vi "SMain.vi"() -> ()   [LabVIEW 2011] (continued)
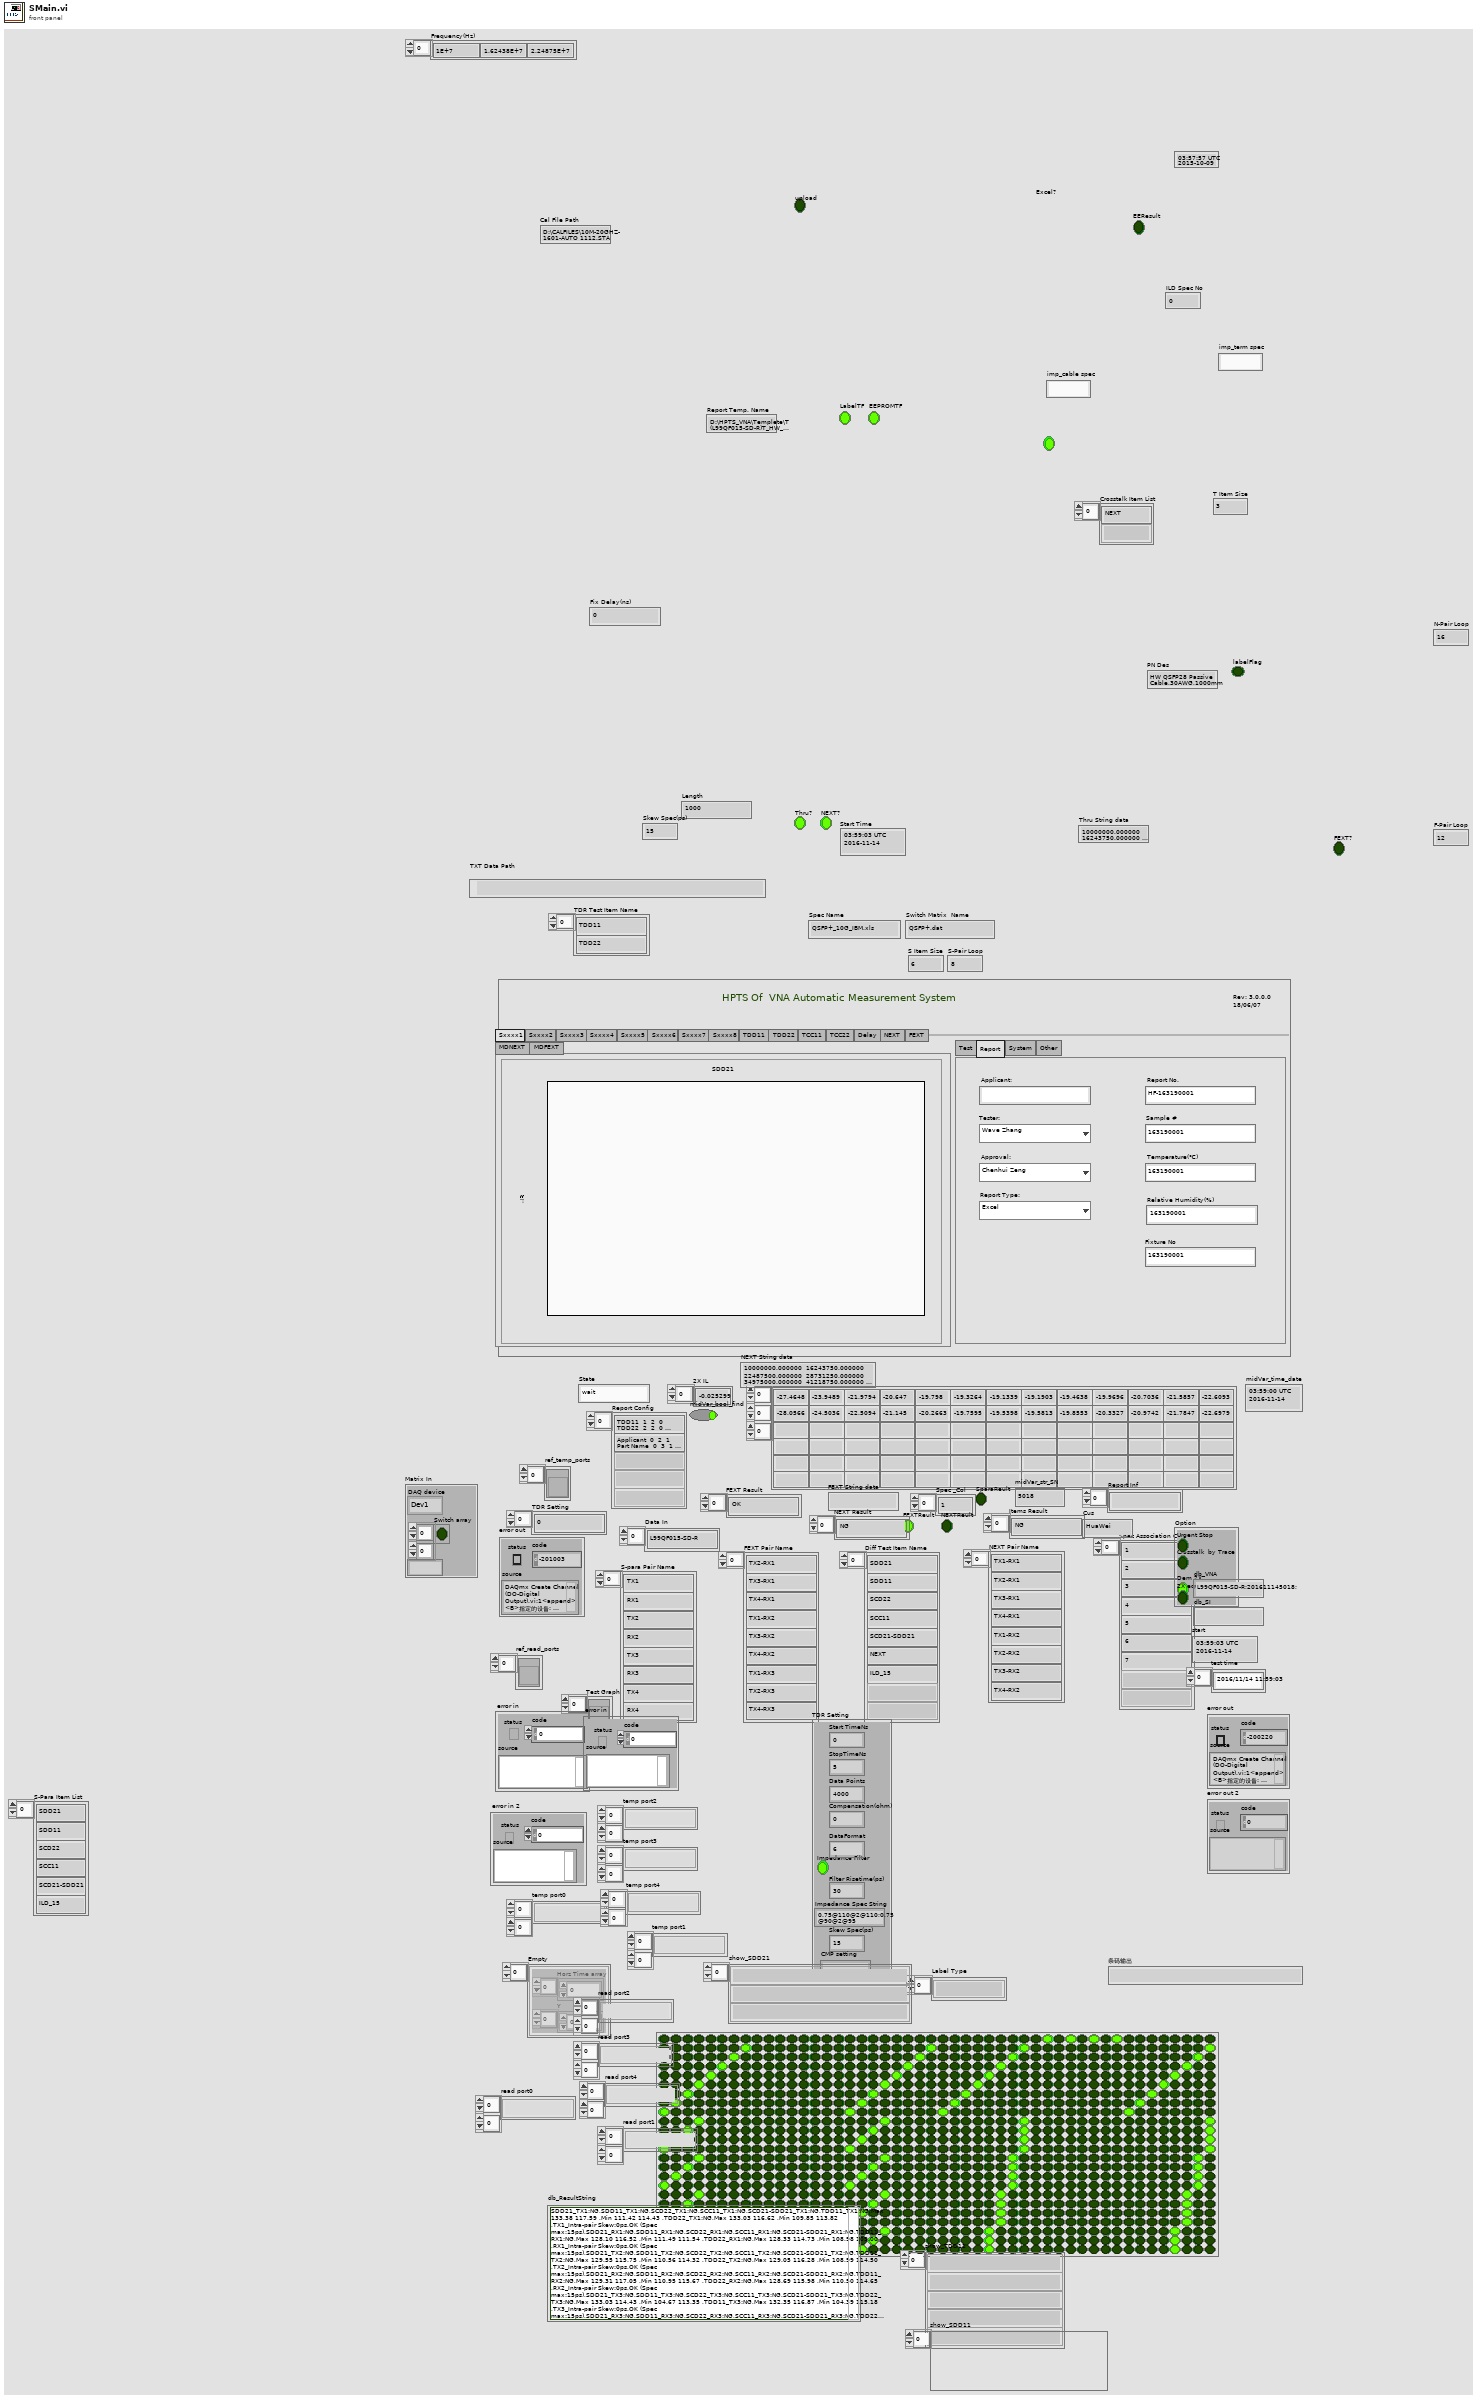
[diagram p1: front panel]
types:
  T1 = typedef "UploadPara.ctl" = cluster{"NetCmdHW":string, "NetPathHW":string, "NetCmdCompress":string, "NetPathCompress1":string, "NetPathCompress2":string, "AlarmDisplay":string, "Synchronous":string, "NetTemppath":string, "NetLocalpath":string}
  T2 = typedef "cluResult.ctl" = cluster{"itemResult":string[], "itemName":string[]}
  T3 = typedef "singleTestParameter.ctl" = cluster{"itemName":string, "testPair":dbl, "chartDisplay?":bool, "spec":cluster{"upper limit":cluster{"dx":dbl[], "dy":dbl[]}, "lowwer limit":cluster{"dx":dbl[], "dy":dbl[]}}, "smooth":cluster{"smooth?":bool, "smoothPoints":dbl}, "Compensation(ohm)":dbl, "Filter Risetime(ps)":dbl, "singlePoint":string[], "offset":dbl[]}
  T4 = typedef "informationIn.ctl" = cluster{"Sample PN: ":string, "SampleSN:":string, "Sparam Test Item":string[], "S-para Pair Name":string[], "Length":string, "Diff Test Item Name":string[], "Diff Test Item Name smooth":string[], "smooth point":dbl, "limitSpec":string[][], "switchIndexOffset":dbl, "testType":enum16{"Loss", "Next", "Fext"}}
  T5 = cluster{"Tab_Graph":refnum<vi>, "Test Graph":refnum<vi>[], "Test Status:":refnum<vi>, "db_ResultString":refnum<vi>}
  T6 = cluster{"Start TimeNs":dbl, "StopTimeNs":dbl, "Data Points":i32, "Compensation(ohm)":dbl, "DataFormat":i16, "Impedance Filter":bool, "Filter Risetime(ps)":dbl, "Impedance Spec String":string, "Skew Spec(ps)":i32, "CMP Setting":string}[]
  T7 = cluster{"start":i32, "length":i32, "p":i32, "H/L":bool}[]
  T8 = cluster{"Server":string, "DB":string, "PSW":string, "User":string}
  T9 = cluster{"auto get refer point":bool, "width1":i32, "width2":i32, "show_TDD11":string[], "show_TDD22":string[], "test time":string[], "show_impspec":string[], "TestResult":bool[], "FileName":string, "FileVersion":string}
  T10 = cluster{"Start TimeNs":dbl, "StopTimeNs":dbl, "Data Points":i32, "Compensation(ohm)":dbl, "DataFormat":i16, "Impedance Filter":bool, "Filter Risetime(ps)":dbl, "Impedance Spec String":string, "Skew Spec(ps)":i32, "CMP Setting":string}
  T11 = cluster{"Urgent Stop":bool, "Crosstalk  by Trace":bool, "Dem 2X":bool, "2X equalize ":bool}
  T12 = cluster{"Start TimeNs":dbl, "StopTimeNs":dbl, "Data Points":i32, "Compensation(ohm)":dbl, "DataFormat":i16, "Impedance Filter":bool, "Filter Risetime(ps)":dbl, "Impedance Spec String":string, "Skew Spec(ps)":i32, "CMP setting":string}
  T13 = cluster{"DAQ device":enum16{"Dev1", "Dev2", "Dev3"}, "Switch array ":bool[][], i32}
  T14 = enum16{"NI PCI-6509", "LX MCU", "LX MCU_40G", "LX MCU_40G_HuaWei"}
  T15 = enum32{"Sxxxx1", "Sxxxx2", "Sxxxx3", "Sxxxx4", "Sxxxx5", "Sxxxx6", "Sxxxx7", "Sxxxx8", "TDD11", "TDD22", "TCC11", "TCC22", "Delay", "NEXT", "FEXT", "MDNEXT", "MDFEXT"}
  T16 = enum16{"Standard Report", "HTML", "Word", "Excel"}
  T17 = enum8{"Enabled", "Disabled", "Disabled and Grayed Out"}
  T18 = typedef "HW_xml.ctl" = cluster{"FileVersion":string, "FileName":string, "test time":string[], "original Path":path, "show_impspec":string[], "usedSN":string, "show_Terminal Point":dbl[], "show_Cable Point":dbl[], "sSpec":T3[], "resultCluster":T2, "customerPN":string}
  T19 = enum32{"invalid app kind", "Development System", "Run Time System", "Student Edition", "Embedded LabVIEW", "Evaluation", "Custom"}
  T20 = cluster{"Urgent Stop":bool, "Crosstalk  by Trace":bool, "Dem 2X":bool, "2x equalize ":bool}
  T21 = cluster{"Demo":bool, "Manual":bool, "Urgent Stop":bool}
  T22 = cluster{"DAQ Device":u16, "Switch array ":bool[][], i32}
  T23 = cluster{"Start TimeNs 2":dbl, "StopTimeNs 2":dbl, "Data Points 2":i32, "Compensation(ohm) 2":dbl, "DataFormat":i16, bool, "Filter Risetime(ps) 2":dbl, "Impedance Spec String 2":string, "Skew Spec(ps) 2":i32, string}
  T24 = cluster{"DAQ Device":u16, "Switch array ":bool[][], "S-Pair Loop":i32}
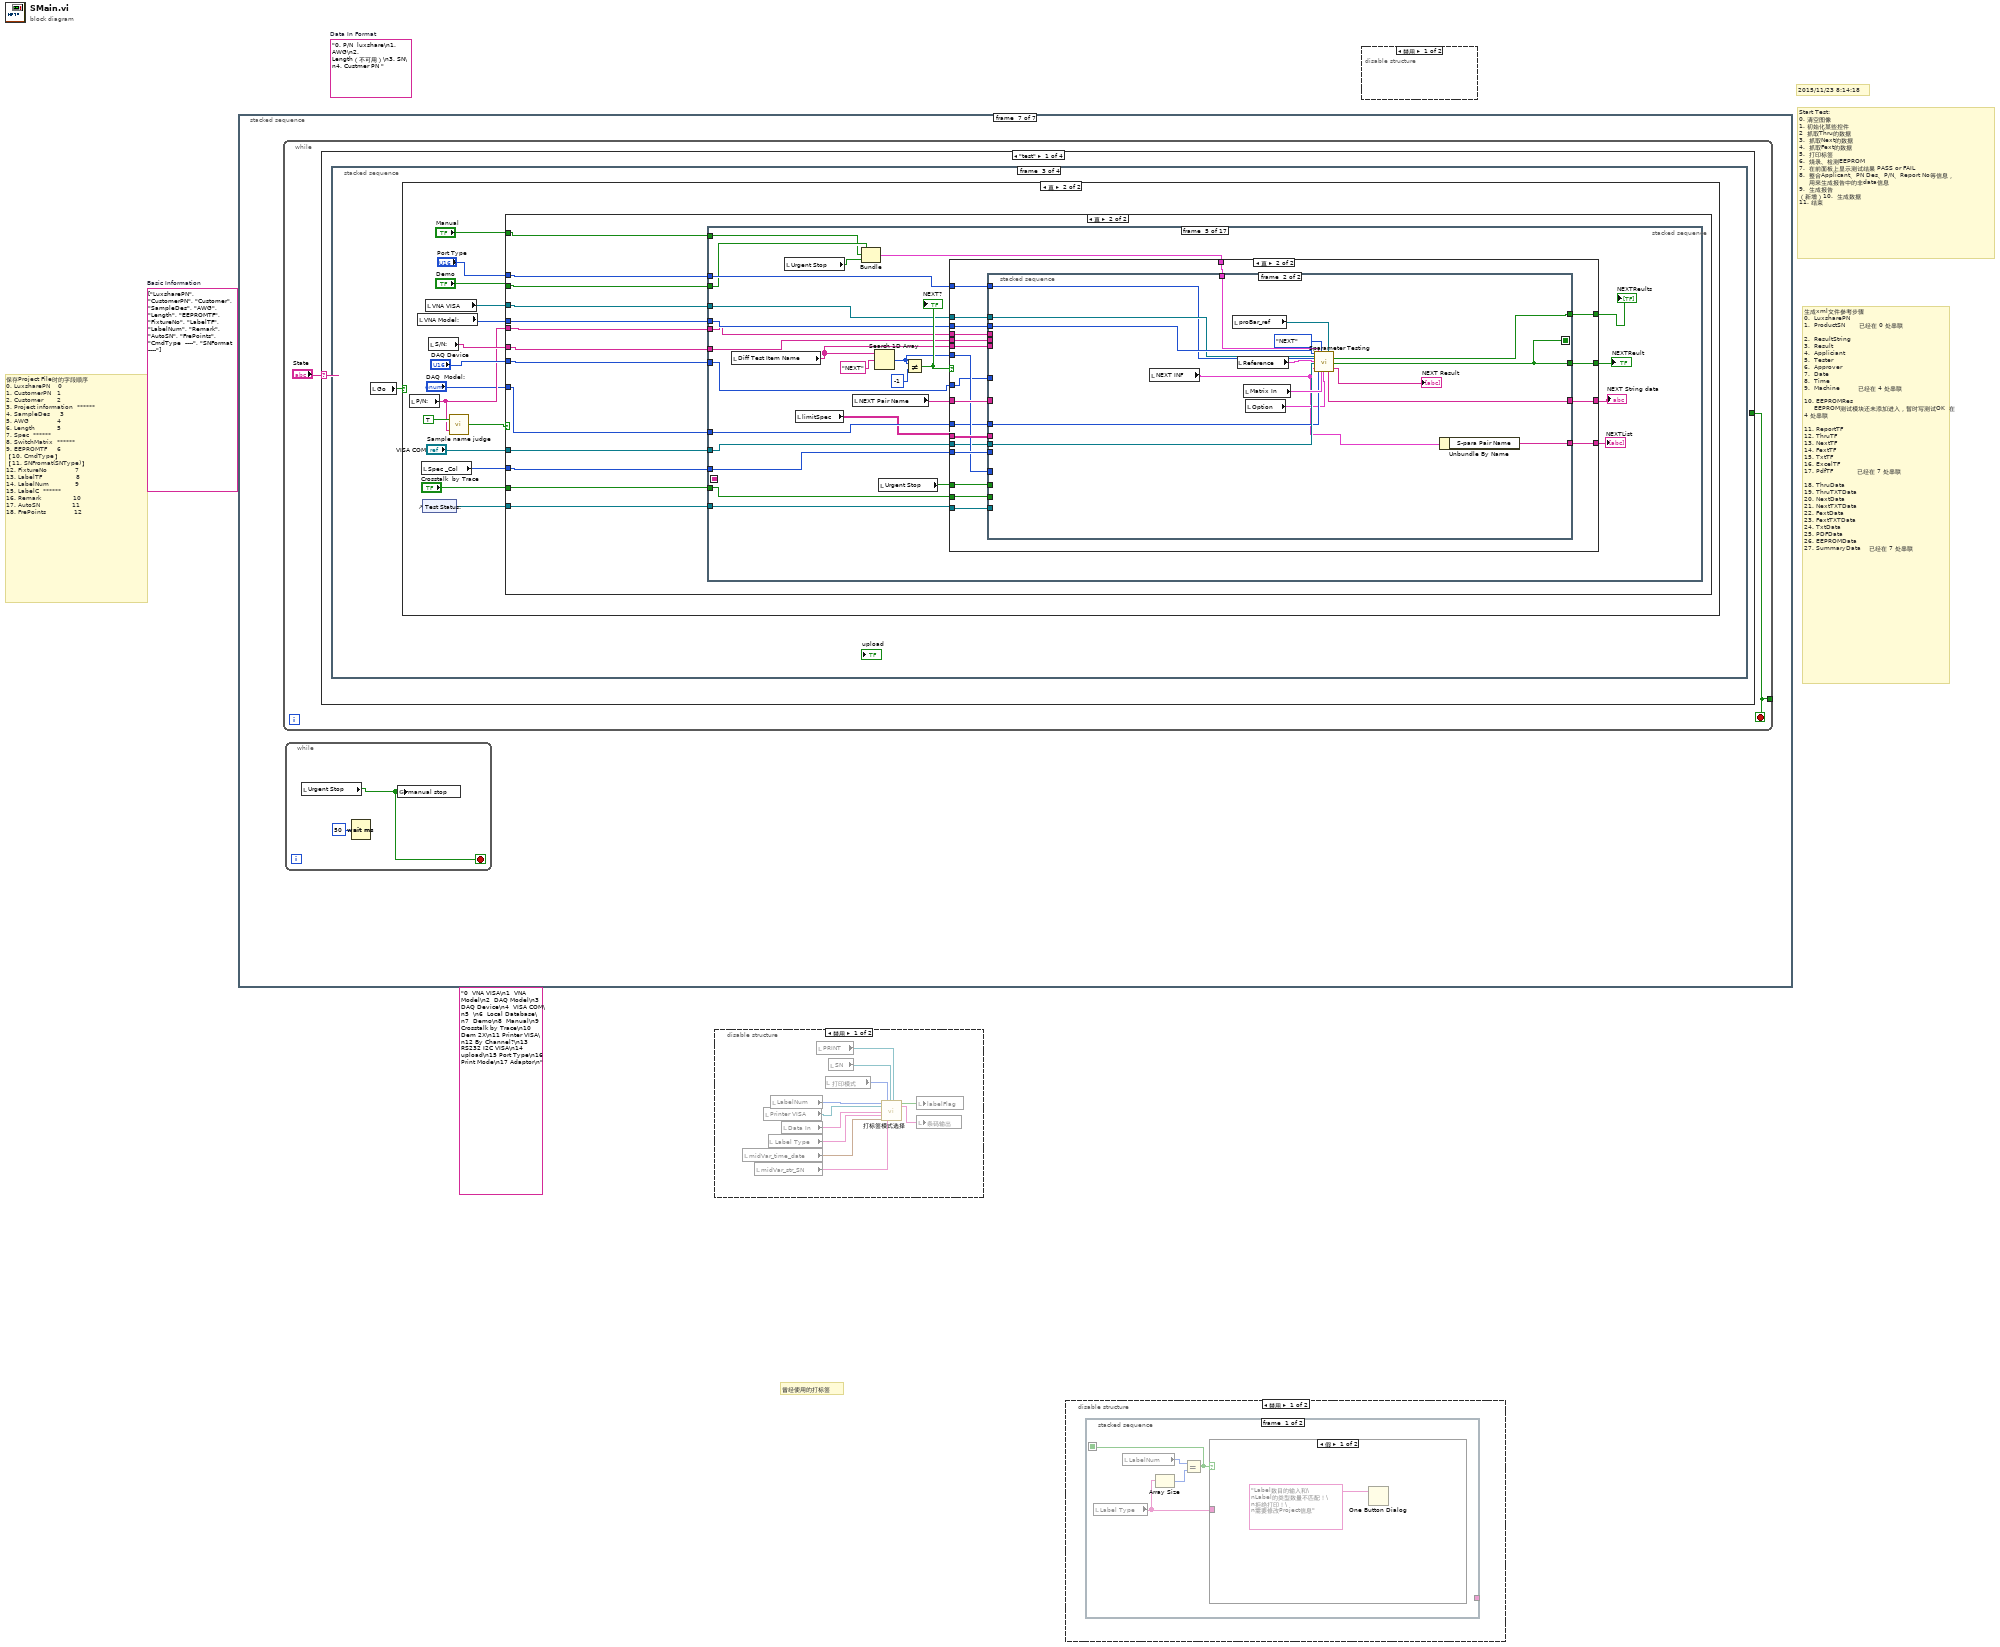
[diagram p0: block diagram]
diagram:
  (unwired) "0  VNA VISA\n1  VNA Model\n2  DAQ Model\n3  DAQ Device\n4  VISA COM\n5  \n6  Local Database\n7  Demo\n8  Manual\n9  Crosstalk by Trace\n10 Dem 2X\n11 Printer VISA\n12 By Channel?\n13 RS232 I2C VISA\n14 upload\n15 Port Type\n16 Print Mode\n17 Adaptor\n"
  (unwired) string[] ["LuxsharePN", "CustomerPN", "Customer", "SampleDes", "AWG", "Length", "EEPROMTF", "FixtureNo", "LabelTF", "LabelNum", "Remark", "AutoSN", "FrePoints", "CmdType  ----", "SNFormat ----"]  # Basic Information
  (unwired) "0. P/N  luxshare\n1. AWG\n2. Length（不可用）\n3. SN\n4. Custmer PN "  # Data In Format
  # "曾经使用的打标签"
  # "保存Project File时的字段顺序\n0. LuxsharePN    0 \n1. CustomerPN   1\n2. Customer       2\n3. Project information  ****** \n4. SampleDes     3\n5. AWG              4\n6. Length           5\n7. Spec  ******\n8. SwitchMatrix  ******  \n9. EEPROMTF     6\n【10. CmdType】           \n【11. SNFromat(SNType)】   \n12. FixtureNo              7\n13. LabelTF                 8\n14. LabelNum             9\n15. LabelC  ******\n16. Remark                10\n17. AutoSN                11\n18. FrePoints              12"
  # "2015/11/23 8:14:18"
  # "生成xml文件参考步骤\n0.  LuxsharePN\n1.  ProductSN       已经在 0 处串联\n\n2.  ResultString     \n3.  Result             \n4.  Appliciant\n5.  Tester\n6.  Approver\n7.  Date \n8.  Time\n9.  Machine         已经在 4 处串联\n\n10. EEPROMRes   \n     EEPROM测试模块还未添加进入，暂时写测试OK  在 4 处串联\n\n11. ReportTF\n12. ThruTF\n13. NextTF\n14. FextTF\n15. TxtTF\n16. ExcelTF\n17. PdfTF            已经在 7 处串联\n\n18. ThruData\n19. ThruTXTData\n20. NextData\n21. NextTXTData\n22. FextData\n23. FextTXTData\n24. TxtData\n25. PDFData\n26. EEPROMData\n27. SummaryData    已经在 7 处串联"
  # "Start Test:\n0. 清空图像\n1. 初始化某些控件 \n2  抓取Thru的数据\n3.  抓取Next的数据\n4.  抓取Fext的数据\n5.  打印标签\n6.  烧录、检测EEPROM\n7.  在前面板上显示测试结果 PASS or FAIL\n8.  整合Applicant、PN Des、P/N、Report No等信息，\n     用来生成报告中的非data信息\n9.  生成报告\n（新增）10.  生成数据 \n11. 结束"
  n1 = stacked-sequence {
    frame #0 {
      n2 = call "AutoUpdate.vi"() -> ()  [unwired: 8 in, 2 out]
      n3 = local write "caliFlag"("" ("caliFlag")) -> ()
    }
    frame #1 {
      # "中间变量"
      n4 = property class="App"() -> ("App.Kind"=w2:T19)  [unwired: 2 in, 2 out]
      n5 = case shown="\"Run Time System\", 默认" w2 {
        frame "Run Time System", Default {
          w4 = ".exe" ("正则表达式")
          n6 = Current VI's Path() -> (path=w7:path)
          n7 = Path To String(path=w7) -> (string=w6:string)
          n8 = xnode "匹配正则表达式"("输入字符串"=w6, "正则表达式"=w4) -> ("匹配之前"=w5:string)  [unwired: 4 in, 4 out]
          n9 = call <vilib>:"Application Directory.vi"() -> ("Application Directory"=w17:path)
          n10 = Build Path(base path=w17, name or relative path="AutoUpdate.xml" ("名称或相对路径")) -> (appended path=w15:path)
          n11 = Concatenate Strings(w5, w4) -> (→"FileName":string)
          n12 = call "xmlConfigRead.vi"("path to XML document"=w15, "XPath expression"="//@Ver") -> ("OutParaArray"=w14:string[])  [unwired: 2 out]
          n13 = Index Array(array=w14, index=4 ("索引")) -> (element=w9:string)
          n14 = call <vilib>:"Trim Whitespace.vi"("string"=w9) -> ("trimmed string"=w12:string)  [unwired: 1 in]
          n15 = String Length(string=w12) -> (length=w11:i32)
          n16 = Equal To 0?(x=w11) -> (x = 0?=w10:bool)
          n17 = case shown="假" w10 {
            tunnel: w9 -> [w130 _]
            tunnel: [w130 "9.9.9.9" ("node text")] -> w8
            frame False {
            }
            frame True {
              n18 = One Button Dialog(message="读取AutoUpdate.xml失败，使用程序默认版本号9.9.9.9" ("消息")) -> ()  [unwired: 1 in, 1 out]
            }
          }
          "FileVersion" <- w8
        }
        frame "Development System" {
          w133 = "DevelopmentSystem" ("FileName")
          n19 = property on="FileName" class="Str"("Value"=w133) -> ()  [unwired: 2 in, 2 out]
          n20 = property on="FileVersion" class="Str"("Value"=w133) -> ()  [unwired: 2 in, 2 out]
        }
      }
    }
    frame #2 {
      w152 = u16 0 items=["Excel", "Excel&PDF"] ("Report Type:")
      w153 = FALSE ("可见")
      w149 = FALSE ("Manual")
      w194 = 2 ("索引")
      w161 = "" ("Sample Description")
      w196 = 0 ("索引")
      n21 = control-ref of="proBar"() -> (→"proBar_ref":refnum<vi>)
      n22 = local write "preStation"("" ("preStation")) -> ()
      n23 = local write "Excel?"(FALSE ("Local Database")) -> ()
      n24 = local write "AutoSN"(FALSE ("AutoSN")) -> ()
      n25 = local write "P/N:"(w161) -> ()
      n26 = property on="Sample Description" class="Str"("Value"="" ("Sample Description"), "Visible"=FALSE ("可见")) -> ()  [unwired: 2 in, 2 out]
      n27 = property on="Tab_System" class="TabCtl (严格)"("Value"=w196) -> ()  [unwired: 2 in, 2 out]
      n28 = property on="Tab_Graph" class="TabCtl (严格)"("Value"=w196) -> ()  [unwired: 2 in, 2 out]
      n29 = property on="Start Test" class="Bool"("DisabledEnum"=w194) -> ()  [unwired: 2 in, 2 out]
      n30 = property on="VNA Initial" class="Bool"("DisabledEnum"=w194) -> ()  [unwired: 2 in, 2 out]
      n31 = local write "Impedance Spec String"(w161) -> ()
      n32 = control-ref of="Delay"() -> (w134:refnum<vi>)
      n33 = control-ref of="TCC11"() -> (w136:refnum<vi>)
      n34 = control-ref of="TCC22"() -> (w135:refnum<vi>)
      n35 = local write "State"("wait" ("state")) -> ()
      n36 = control-ref of="MDNEXT"() -> (w137:refnum<vi>)
      n37 = control-ref of="PASS"() -> (w206:refnum<vi>)
      n38 = control-ref of="PASS"() -> (w205:refnum<vi>)
      n39 = control-ref of="Test Graph3"() -> (w204:refnum<vi>)
      n40 = control-ref of="Test Graph4"() -> (w203:refnum<vi>)
      n41 = control-ref of="Test Graph5"() -> (w202:refnum<vi>)
      n42 = control-ref of="Test Graph6"() -> (w201:refnum<vi>)
      n43 = control-ref of="Test Graph7"() -> (w200:refnum<vi>)
      n44 = control-ref of="Test Graph8"() -> (w199:refnum<vi>)
      n45 = control-ref of="TDD11 Graph"() -> (w186:refnum<vi>)
      n46 = control-ref of="TDD22 Graph"() -> (w185:refnum<vi>)
      n47 = control-ref of="Next"() -> (w184:refnum<vi>)
      n48 = control-ref of="Test Graph10"() -> (w183:refnum<vi>)
      n49 = control-ref of="MDFEXT"() -> (w138:refnum<vi>)
      n50 = local write "Current Testing Label/当前测试条码"("") -> ()
      n51 = Build Array(w206, w205, w204, w203, w202, w201, w200, w199, w186, w185, w136, w135, w134, w184, w183, w138, w137) -> (w198:refnum<vi>[])
      "Test Graph" <- w198
      n52 = property on="Result" class="Str"("Visible"=FALSE ("可见"), "Value"="Testing..." ("Result"), "DisabledEnum"=1, "Text.BGColor"=u32 16777216) -> ()  [unwired: 2 in, 2 out]
      n53 = local write "Demo"(w149) -> ()
      n54 = local write "Dem 2X"(w149) -> ()
      n55 = local write "Manual"(w149) -> ()
      n56 = local write "Excel?"(w149) -> ()
      n57 = property on="Urgent Stop" class="Bool (严格)"("DisabledEnum"=0 ("索引")) -> ()  [unwired: 2 in, 2 out]
      n58 = property on="Report Type:" class="Ring (严格)"("Value"=w152) -> ()  [unwired: 2 in, 2 out]
      n59 = property on="Start Page" class="DigNum (严格)"("Visible"=w153) -> ()  [unwired: 2 in, 2 out]
      n60 = property on="End Page" class="DigNum (严格)"("Visible"=w153) -> ()  [unwired: 2 in, 2 out]
      n61 = local write "Local Database"(w149) -> ()
      n62 = local write "Auto Count:"(w149) -> ()
      n63 = local write "Crosstalk  by Trace"(w149) -> ()
      n64 = local write "Urgent Stop"(w149) -> ()
      n65 = for {
        tunnel: w198 -> [w240] mode=indexing
        tunnel: "Empty" -> [w239]
        n66 = property class="XYGraph (严格)"(reference=w240, "Value"=w239, "Caption.Visible"=FALSE ("标题.可见")) -> ()  [unwired: 1 in, 2 out]
      }
      n67 = call "运行批处理.vi"() -> ()  [unwired: 12 in]
      n68 = local write "Use Counts?"(TRUE ("Use Counts?")) -> ()
      n69 = local read "VISA COM"() -> (w160:refnum<visa-resource-name>)
      n70 = local read "DAQ Device"() -> (w158:u16)
      n71 = stacked-sequence {
        frame #0 {
          n72 = control-ref of="temp port0"() -> (w212:refnum<vi>)
          n73 = control-ref of="temp port1"() -> (w211:refnum<vi>)
          n74 = control-ref of="temp port2"() -> (w210:refnum<vi>)
          n75 = control-ref of="temp port3"() -> (w209:refnum<vi>)
          n76 = control-ref of="temp port4"() -> (w208:refnum<vi>)
          n77 = Build Array(w212, w211, w210, w209, w208) -> (→"ref_temp_ports":refnum<vi>[])
        }
        frame #1 {
          n78 = control-ref of="read port0"() -> (w218:refnum<vi>)
          n79 = control-ref of="read port1"() -> (w217:refnum<vi>)
          n80 = control-ref of="read port2"() -> (w216:refnum<vi>)
          n81 = control-ref of="read port3"() -> (w215:refnum<vi>)
          n82 = control-ref of="read port4"() -> (w214:refnum<vi>)
          n83 = Build Array(w218, w217, w216, w215, w214) -> (→"ref_read_ports":refnum<vi>[])
        }
      }
      n84 = local read "Manual"() -> (w156:bool)
      n85 = local read "DAQ  Model:"() -> (w159:T14)
      n86 = local read "Demo"() -> (w155:bool)
      n87 = Format Date/Time String(time format string (%c)="%#j") -> (date/time string=w189:string)  [unwired: 2 in]
      n88 = String Length(string=w189) -> (length=w190:i32)
      n89 = Or(x=w156, y=w155) -> (x .or. y?=w157:bool)
      n90 = call <vilib>:"Application Directory.vi"() -> ("Application Directory"=w173:path)
      n91 = case shown="2" w190 {
        tunnel: w189 -> [w232 w236 w237]
        tunnel: [w231 w235 w237] -> w188
        frame 1, Default {
          n92 = Concatenate Strings("00" ("字符串"), w232) -> (w231:string)
        }
        frame 2 {
          n93 = Concatenate Strings("0" ("字符串"), w236) -> (w235:string)
        }
        frame 3 {
        }
      }
      n94 = Build Path(base path=w173, name or relative path="database\\inf.txt" ("名称或相对路径")) -> (appended path=w171:path)
      n95 = case shown="假" w157 {
        tunnel: w158 -> [w221 _]
        tunnel: w159 -> [w220 _]
        tunnel: w160 -> [w219 _]
        frame False {
          n96 = case shown="\"LX MCU\"" w220 {
            tunnel: w221 -> [w226 _ _]
            tunnel: w219 -> [_ w228 w230]
            frame "NI PCI-6509", Default {
              n97 = local read "Switch array"() -> (w224:bool[][])
              n98 = call "6509 simple.vi"("error in"="error in", "index (row)"=i8 79, "array input: P0-P1-P2-P3-P4-P5"=w224, "DAQ device"=w226) -> ("error out"=→"error out":errorcluster)  [unwired: 3 in]
            }
            frame "LX MCU" {
              w227 = u16 1 items=["Testing", "Close All"] ("Function")
              n99 = call "MCU Switch Control.vi"("Function"=w227, "VISA"=w228) -> ()  [unwired: 9 in, 1 out]
            }
            frame "LX MCU_40G" {
              w229 = u16 1 items=["Testing", "Close All"] ("Function")
              n100 = call "40G MCU Switch Control.vi"("Function"=w229, "VISA"=w230) -> ()  [unwired: 9 in, 1 out]
            }
          }
        }
        frame True {
        }
      }
      n101 = call-poly <vilib>:"Read From Spreadsheet File.vi"("file path (dialog if empty)"=w171) -> ("all rows"=w170:string[][])  [unwired: 6 in, 4 out]
      n102 = Delete From Array(array=w170, index (row)=0 ("索引 (行)")) -> (array with subset deleted=w168:string[][])  [unwired: 2 in, 1 out]
      n103 = Format Date/Time String(time format string (%c)="%#y") -> (date/time string=w193:string)  [unwired: 2 in]
      n104 = Index Array(array=w168, index (col) #1=6 ("禁用的索引 (列)"), index (col) #2=7 ("索引 (列)")) -> (element #1=w165:string[], element #2=w164:string[])  [unwired: 2 in]
      n105 = Concatenate Strings(w193, w188, "0001" ("字符串")) -> (w174:string)
      n106 = call "Delete empty element from array.vi"("Array In"=w165) -> ("Array out"=w163:string[])  [unwired: 26 in]
      n107 = local write "Sample #"(w174) -> ()
      n108 = call "Delete empty element from array.vi"("Array In"=w164) -> ("Array out"=w162:string[])  [unwired: 26 in]
      n109 = local write "S/N:"(w174) -> ()
      n110 = Concatenate Strings("HF-" ("字符串"), w174) -> (w176:string)
      n111 = property on="Approval:" class="Ring (严格)"("Strings []"=w162) -> ()  [unwired: 2 in, 2 out]
      n112 = property on="Tester:" class="Ring (严格)"("Strings []"=w163) -> ()  [unwired: 2 in, 2 out]
      n113 = local write "Test Status:"("Please do full calibration for VNA with E-Cal module before start test!\nThen, click \"VNA initial\" buttom to recall calibration file!" ("Test Status:")) -> ()
      n114 = local write "Report No."(w176) -> ()
      "proBar" <- u8 0 ("proBar")
      "Go" <- FALSE ("show_bool_checkResult")
      "UseAge" <- u8 0 ("寿命")
      "Used" <- u8 0 ("已用")
      "strFSN 原始SN" <- "" ("strFSN 原始SN")
    }
    frame #3 {
      (unwired) string[][] [["VNA VISA", "E5071C"], ["VNA Model", "E5071C"], ["DAQ Model", "NI PCI-6509"], ["DAQ Device", "Dev1"], ["VISA COM", "COM4"], ["checkBeforeTest", "FALSE"], ["Local Database", "TRUE"], ["Demo", "TRUE"], ["Manual", "FALSE"], ["Crosstalk by Trace", "FALSE"], ["Dem 2X", "FALSE"], ["By Channel?", "FALSE"], ["Print VISA", "USB0::0x0A5F::0x00AB::JJL045601::RAW"], ["RS232 I2C VISA", "COM1"], ["Data UpLoad", "FALSE"], ["Port Type", "1"], ["Print Mode", "IT Print"], ["Adaptor", "RS232 - IIC"]] ("all rows")
      (unwired) "0  VNA VISA\n1  VNA Model\n2  DAQ Model\n3  DAQ Device\n4  VISA COM\n5  \n6  Local Database\n7  Demo\n8  Manual\n9  Crosstalk by Trace\n10 Dem 2X\n11 Printer VISA\n12 By Channel?\n13 RS232 I2C VISA\n14 upload\n15 Port Type\n16 Print Mode\n17 Adaptor\n"
      # "加载主页面配置信息"
      n115 = call <vilib>:"Application Directory.vi"() -> ("Application Directory"=w245:path)
      n116 = Build Path(base path=w245, name or relative path="database\\initializeConfig.txt" ("名称或相对路径")) -> (appended path=w243:path)
      n117 = call <vilib>:"Check if File or Folder Exists.vi"("path"=w243) -> ("file or folder exists?"=w242:bool, "dup path"=w241:path)  [unwired: 8 in, 1 out]
      n118 = case shown="真" w242 {
        tunnel: w241 -> [w307 w345]
        frame False {
          w251 = string[][] [["VNA VISA", "E5071C"], ["VNA Model", "E5071C"], ["DAQ Model", "NI PCI-6509"], ["DAQ Device", "Dev1"], ["VISA COM", "COM4"], ["checkBeforeTest", "FALSE"], ["Local Database", "TRUE"], ["Demo", "TRUE"], ["Manual", "FALSE"], ["Crosstalk by Trace", "FALSE"], ["Dem 2X", "FALSE"], ["By Channel?", "FALSE"], ["Print VISA", "USB0::0x0A5F::0x00AB::JJL045601::RAW"], ["RS232 I2C VISA", "COM1"], ["Data UpLoad", "FALSE"], ["Port Type", "1"], ["Print Mode", "IT Print"], ["Adaptor", "RS232 - IIC"], ["Use Counts", "TRUE"], ["RS232 I2C VISA Counts", "COM1"]] ("all rows")
          n119 = Index Array(array=w251, index (col)=1 ("禁用的索引 (列)")) -> (element=w261:string[])  [unwired: 1 in]
          n120 = call-poly <vilib>:"Write To Spreadsheet File.vi"("2D data"=w251, "file path (dialog if empty)"=w307) -> ()  [unwired: 6 in, 1 out]
          n121 = Index Array(array=w261, index #1=0 ("索引"), index #6=5 ("索引"), index #11=10 ("索引"), index #16=15 ("索引")) -> (element #1=w268:string, element #2=w306:string, element #3=w304:string, element #4=w302:string, element #5=w301:string, element #6=w293:string, element #7=w292:string, element #8=w285:string, element #9=w281:string, element #10=w277:string, element #11=w275:string, element #12=w271:string, element #13=w270:string, element #14=w269:string, element #15=w264:string, element #16=w257:string, element #17=w255:string, element #18=w252:string, element #19=w248:string, element #20=w246:string)  [unwired: 16 in]
          n122 = local write "RS232 I2C Counts"(w246) -> ()
          n123 = case shown="\"IT Print\", 默认" w255 {
            tunnel: [0 1] -> w254
            frame "IT Print", Default {
            }
            frame "EE Print" {
            }
          }
          n124 = Decimal String To Number(string=w257) -> (number=w263:i32)  [unwired: 2 in, 1 out]
          n125 = To Upper Case(1:w277) -> (0:w284:string)
          n126 = To Upper Case(1:w271) -> (0:w274:string)
          n127 = To Upper Case(1:w275) -> (0:w279:string)
          n128 = To Upper Case(1:w293) -> (0:w298:string)
          n129 = local write "Port Type"(w263) -> ()
          n130 = To Upper Case(1:w292) -> (0:w295:string)
          n131 = Equal?(x=w284, y="TRUE") -> (x = y?=w282:bool)
          n132 = Equal?(x=w274, y="TRUE") -> (x = y?=w272:bool)
          n133 = Equal?(x=w279, y="TRUE") -> (x = y?=w278:bool)
          n134 = property on="VNA VISA" class="VISAName"("Value"=w268) -> ()  [unwired: 2 in, 2 out]
          n135 = Equal?(x=w298, y="TRUE") -> ()  [unwired: 1 out]
          n136 = Equal?(x=w295, y="TRUE") -> (x = y?=w294:bool)
          n137 = local write "打印模式"(w254) -> ()
          n138 = case shown="\"N5230A(C)\"" w306 {
            tunnel: [0 1 2] -> w305
            frame "E5071C", Default {
            }
            frame "N5230A(C)" {
            }
            frame "N5224A" {
            }
          }
          n139 = case shown="\"Dev3\"" w302 {
            tunnel: [0 1 2] -> w303
            frame "Dev1", Default {
            }
            frame "Dev2" {
            }
            frame "Dev3" {
            }
          }
          n140 = case shown="\"NI PCI-6509\", 默认" w304 {
            tunnel: [0 1] -> w258
            frame "NI PCI-6509", Default {
            }
            frame "LX MCU" {
            }
          }
          n141 = local write "Crosstalk  by Trace"(w282) -> ()
          n142 = local write "Local Database"(w294) -> ()
          n143 = local write "Dem 2X"(w278) -> ()
          n144 = local write "By Channel?"(w272) -> ()
          n145 = case shown="\"RS232 - IIC\", 默认" w252 {
            tunnel: [0 1] -> w253
            frame "RS232 - IIC", Default {
            }
            frame "LUXSHARE - IIC" {
            }
          }
          n146 = To Upper Case(1:w264) -> (0:w266:string)
          n147 = local write "RS232 I2C VISA"(w269) -> ()
          n148 = local write "VNA Model:"(w305) -> ()
          n149 = local write "Printer VISA"(w270) -> ()
          n150 = local write "DAQ  Model:"(w258) -> ()
          n151 = local write "DAQ Device"(w303) -> ()
          n152 = Equal?(x=w266, y="TRUE") -> (x = y?=w265:bool)
          n153 = local write "VISA COM"(w301) -> ()
          n154 = To Upper Case(1:w285) -> (0:w291:string)
          n155 = To Upper Case(1:w281) -> (0:w288:string)
          n156 = Equal?(x=w291, y="TRUE") -> (x = y?=w287:bool)
          n157 = Equal?(x=w288, y="TRUE") -> (x = y?=w286:bool)
          n158 = local write "upload"(w265) -> ()
          n159 = local write "Demo"(w287) -> ()
          n160 = local write "Manual"(w286) -> ()
          n161 = local write "Adaptor:"(w253) -> ()
          n162 = case shown="1" w258 {
            tunnel: [2 0] -> w260
            tunnel: [0 2] -> w259
            frame 0, Default {
            }
            frame 1 {
            }
          }
          n163 = disable-structure shown="禁用" {
            disable-tunnel: w265 -> [w309 _]
            frame Disabled {
              w310 = "Data UpLoad" ("项标识符")
              n164 = Current VI's Menubar() -> (w313:refnum<k9>)
              n165 = Get Menu Item Info(7:w310, 11:w313) -> (2:w311:string, 3:w312:refnum<k9>)  [unwired: 1 in, 5 out]
              n166 = Set Menu Item Info(6:w309, 7:w310, 9:TRUE ("已启用"), 10:w311, 11:w312) -> ()  [unwired: 2 in, 2 out]
            }
            frame Enabled {
            }
          }
          n167 = To Upper Case(1:w248) -> (0:w250:string)
          n168 = Equal?(x=w250, y="TRUE") -> (x = y?=w247:bool)
          n169 = property on="DAQ Device" class="Ring (严格)"("DisabledEnum"=w259) -> ()  [unwired: 2 in, 2 out]
          n170 = property on="VISA COM" class="VISAName"("DisabledEnum"=w260) -> ()  [unwired: 2 in, 2 out]
          n171 = local write "Use Counts?"(w247) -> ()
        }
        frame True {
          n172 = call-poly <vilib>:"Read From Spreadsheet File.vi"("file path (dialog if empty)"=w345) -> ("all rows"=w391:string[][])  [unwired: 6 in, 4 out]
          n173 = Index Array(array=w391, index (col)=1 ("禁用的索引 (列)")) -> (element=w389:string[])  [unwired: 1 in]
          n174 = Index Array(array=w389, index #1=0 ("索引"), index #6=5 ("索引"), index #11=10 ("索引"), index #16=15 ("索引")) -> (element #1=w351:string, element #2=w388:string, element #3=w386:string, element #4=w384:string, element #5=w383:string, element #6=w375:string, element #7=w374:string, element #8=w367:string, element #9=w363:string, element #10=w359:string, element #11=w357:string, element #12=w353:string, element #13=w335:string, element #14=w352:string, element #15=w347:string, element #16=w340:string, element #17=w337:string, element #18=w336:string, element #19=w331:string, element #20=w330:string)  [unwired: 16 in]
          n175 = local write "RS232 I2C Counts"(w330) -> ()
          n176 = case shown="\"IT Print\", 默认" w337 {
            tunnel: [0 1] -> w339
            frame "IT Print", Default {
            }
            frame "EE Print" {
            }
          }
          n177 = Decimal String To Number(string=w340) -> (number=w346:i32)  [unwired: 2 in, 1 out]
          n178 = local write "Port Type"(w346) -> ()
          n179 = To Upper Case(1:w359) -> (0:w366:string)
          n180 = To Upper Case(1:w353) -> (0:w356:string)
          n181 = To Upper Case(1:w357) -> (0:w361:string)
          n182 = To Upper Case(1:w375) -> (0:w380:string)
          n183 = To Upper Case(1:w374) -> (0:w377:string)
          n184 = Equal?(x=w366, y="TRUE") -> (x = y?=w364:bool)
          n185 = Equal?(x=w356, y="TRUE") -> (x = y?=w354:bool)
          n186 = Equal?(x=w361, y="TRUE") -> (x = y?=w360:bool)
          n187 = property on="VNA VISA" class="VISAName"("Value"=w351) -> ()  [unwired: 2 in, 2 out]
          n188 = Equal?(x=w380, y="TRUE") -> ()  [unwired: 1 out]
          n189 = Equal?(x=w377, y="TRUE") -> (x = y?=w376:bool)
          n190 = local write "打印模式"(w339) -> ()
          n191 = case shown="\"N5224A\"" w388 {
            tunnel: [0 1 2] -> w387
            frame "E5071C", Default {
            }
            frame "N5230A(C)" {
            }
            frame "N5224A" {
            }
          }
          n192 = case shown="\"Dev3\"" w384 {
            tunnel: [0 1 2] -> w385
            frame "Dev1", Default {
            }
            frame "Dev2" {
            }
            frame "Dev3" {
            }
          }
          n193 = case shown="\"NI PCI-6509\", 默认" w386 {
            tunnel: [0 1] -> w342
            frame "NI PCI-6509", Default {
            }
            frame "LX MCU" {
            }
          }
          n194 = local write "Crosstalk  by Trace"(w364) -> ()
          n195 = local write "Local Database"(w376) -> ()
          n196 = local write "Dem 2X"(w360) -> ()
          n197 = local write "By Channel?"(w354) -> ()
          n198 = case shown="\"LUXSHARE - IIC\"" w336 {
            tunnel: [0 1] -> w338
            frame "RS232 - IIC", Default {
            }
            frame "LUXSHARE - IIC" {
            }
          }
          n199 = To Upper Case(1:w347) -> (0:w349:string)
          n200 = local write "RS232 I2C VISA"(w352) -> ()
          n201 = local write "VNA Model:"(w387) -> ()
          n202 = local write "Printer VISA"(w335) -> ()
          n203 = local write "DAQ  Model:"(w342) -> ()
          n204 = local write "DAQ Device"(w385) -> ()
          n205 = Equal?(x=w349, y="TRUE") -> (x = y?=w348:bool)
          n206 = local write "VISA COM"(w383) -> ()
          n207 = To Upper Case(1:w367) -> (0:w373:string)
          n208 = To Upper Case(1:w363) -> (0:w370:string)
          n209 = local write "upload"(w348) -> ()
          n210 = Equal?(x=w373, y="TRUE") -> (x = y?=w369:bool)
          n211 = Equal?(x=w370, y="TRUE") -> (x = y?=w368:bool)
          n212 = local write "Adaptor:"(w338) -> ()
          n213 = local write "Demo"(w369) -> ()
          n214 = local write "Manual"(w368) -> ()
          n215 = case shown="1" w342 {
            tunnel: [2 0] -> w344
            tunnel: [0 2] -> w343
            frame 0, Default {
            }
            frame 1 {
            }
          }
          n216 = disable-structure shown="禁用" {
            disable-tunnel: w348 -> [w393 _]
            frame Disabled {
              w394 = "Data UpLoad" ("项标识符")
              n217 = Current VI's Menubar() -> (w397:refnum<k9>)
              n218 = Get Menu Item Info(7:w394, 11:w397) -> (2:w395:string, 3:w396:refnum<k9>)  [unwired: 1 in, 5 out]
              n219 = Set Menu Item Info(6:w393, 7:w394, 9:TRUE ("已启用"), 10:w395, 11:w396) -> ()  [unwired: 2 in, 2 out]
            }
            frame Enabled {
            }
          }
          n220 = property on="DAQ Device" class="Ring (严格)"("DisabledEnum"=w343) -> ()  [unwired: 2 in, 2 out]
          n221 = property on="VISA COM" class="VISAName"("DisabledEnum"=w344) -> ()  [unwired: 2 in, 2 out]
          n222 = To Upper Case(1:w331) -> (0:w332:string)
          n223 = Equal?(x=w332, y="TRUE") -> (x = y?=w334:bool)
          n224 = local write "Use Counts?"(w334) -> ()
        }
      }
    }
    frame #4 {
      w433 = T8 {"Server"="", "DB"="", "PSW"="", "User"=""}  # DBSet
      n225 = call <vilib>:"Application Directory.vi"() -> ("Application Directory"=w490:path)
      n226 = Build Path(base path=w490, name or relative path="Database" ("名称或相对路径")) -> (appended path=w488:path)
      n227 = call <vilib>:"Application Directory.vi"() -> ("Application Directory"=w500:path)
      n228 = call <vilib>:"Application Directory.vi"() -> ("Application Directory"=w518:path)
      n229 = call <vilib>:"Check if File or Folder Exists.vi"("path"=w488) -> ("file or folder exists?"=w487:bool, "dup path"=w486:path)  [unwired: 8 in, 1 out]
      n230 = Build Path(base path=w518, name or relative path="EEPROM Code\\tempory_folder" ("名称或相对路径")) -> (appended path=w510:path)
      n231 = Build Path(base path=w500, name or relative path="Database" ("名称或相对路径")) -> (appended path=w498:path)
      n232 = case shown="假" w487 {
        tunnel: w486 -> [w547 w548]
        tunnel: [w546 w548] -> w485
        frame False {
          n233 = Create Folder(path (use dialog)=w547) -> (created path=w546:path)  [unwired: 2 in, 2 out]
        }
        frame True {
        }
      }
      n234 = call <vilib>:"Check if File or Folder Exists.vi"("path"=w510) -> ("file or folder exists?"=w509:bool, "dup path"=w508:path)  [unwired: 8 in, 1 out]
      n235 = call <vilib>:"Check if File or Folder Exists.vi"("path"=w498) -> ("file or folder exists?"=w497:bool, "dup path"=w496:path)  [unwired: 8 in, 1 out]
      n236 = case shown="假" w509 {
        tunnel: w508 -> [w571 w572]
        tunnel: [w570 w572] -> w507
        frame False {
          n237 = Create Folder(path (use dialog)=w571) -> (created path=w570:path)  [unwired: 2 in, 2 out]
        }
        frame True {
        }
      }
      n238 = case shown="假" w497 {
        tunnel: w496 -> [w566 w567]
        tunnel: [w565 w567] -> w495
        frame False {
          n239 = Create Folder(path (use dialog)=w566) -> (created path=w565:path)  [unwired: 2 in, 2 out]
        }
        frame True {
        }
      }
      n240 = Build Path(base path=w485, name or relative path="FigoConfig.xml" ("名称或相对路径")) -> (appended path=w483:path)
      n241 = call <vilib>:"Check if File or Folder Exists.vi"("path"=w483) -> ("file or folder exists?"=w482:bool, "dup path"=w458:path)  [unwired: 8 in, 1 out]